vi "UHR-Fleezers Control (host) - 12.4.vi"() -> ()   [LabVIEW 2012] (continued)
                n1986 = Negate(x=w2940) -> (-x=w2941:dbl)
                n1987 = local read "Initial Y"() -> (w2947:dbl)
                n1988 = Multiply(x=w2929, y=w2938) -> (x*y=w2948:dbl)
                n1989 = Divide "X half step offset"(x=w2926, y=2.0) -> (x/y=w2934:dbl)
                n1990 = Divide "X V/pix"(x=w2926, y=w2937) -> (x/y=w2936:dbl)
                n1991 = Multiply(x=w2926, y=w2931) -> (x*y=w2943:dbl)
                n1992 = Compound Arithmetic op=ADD(w2941, w2948, w2947) -> (w2918:dbl)
                "Pointer Y (V)" <- w2918
                n1993 = Multiply(x=w2936, y=w2930) -> (x*y=w2945:dbl)
                n1994 = Negate(x=w2934) -> (-x=w2933:dbl)
                n1995 = local read "Initial X"() -> (w2946:dbl)
                n1996 = Negate(x=w2945) -> (-x=w2944:dbl)
                n1997 = Compound Arithmetic op=ADD(w2933, w2943, w2946, w2944) -> (w2919:dbl)
                "Pointer X (V)" <- w2919
                n1998 = case shown="True" "Set High F Confocal Spot (X-Y)" {
                  tunnel: w2919 -> [_ w2949]
                  tunnel: w2918 -> [_ w2950]
                  frame False {
                  }
                  frame True {
                    "Confocal Y 2 (V)" <- w2950
                    "Confocal X 2 (V)" <- w2949
                  }
                }
                n1999 = Or(x="Set X Only", y="Set Confocal Spot (X-Y)") -> (x .or. y?=w2922:bool)
                n2000 = Or(x="Set Confocal Spot (X-Y)", y="Set Y Only") -> (x .or. y?=w2921:bool)
                n2001 = case shown="True" w2922 {
                  tunnel: w2919 -> [_ w2951]
                  frame False {
                  }
                  frame True {
                    n2002 = property on="AO2" class="Slide (strict)"("Val(Sgnl)"=w2951) -> ()  [unwired: 2 in, 2 out]
                    "Confocal X 1 (V)" <- w2951
                  }
                }
                n2003 = case shown="True" w2921 {
                  tunnel: w2918 -> [_ w2952]
                  frame False {
                  }
                  frame True {
                    n2004 = property on="AO1" class="Slide (strict)"("Val(Sgnl)"=w2952) -> ()  [unwired: 2 in, 2 out]
                    "Confocal Y 1 (V)" <- w2952
                  }
                }
                n2005 = local write "Set High F Confocal Spot (X-Y)"(w2917) -> ()
                n2006 = local write "Set Confocal Spot (X-Y)"(w2917) -> ()
                n2007 = local write "Set X Only"(w2917) -> ()
                n2008 = local write "Set Y Only"(w2917) -> ()
              }
            }
          }
          frame 3 {
            n2009 = local read "BD 2 Frequency 1 (MHz)"() -> (w2953:dbl)
            n2010 = local read "BD 1 Frequency 1 (MHz)"() -> (w2954:dbl)
            n2011 = local write "Manipulating Trap"(TRUE ("Manipulating Trap")) -> ()
            n2012 = local write "Coords"(T7 {"Horizontal"=0, "Vertical"=0} ("Coords")) -> ()
            n2013 = while {
              tunnel: w2959 -> [w2964]
              tunnel: w2957 -> [w2963]
              tunnel: w2955 -> [w2962]
              tunnel: w2954 -> [w2961]
              tunnel: w2953 -> [w2960]
              stop <- w2965 stop-if-true
              n2014 = event shown="[0] \"Pane\": Mouse Move" {
                selector: _ -> [_ _]
                dyn-events: _ -> [_ _]
                timeout: _ -> [_ _]
                tunnel: ["Force Manip Abort" w3029] -> w2965
                tunnel: w2964 -> [w2972 _]
                tunnel: w2963 -> [w2970 _]
                tunnel: w2962 -> [w2969 _]
                tunnel: w2961 -> [w2968 _]
                tunnel: w2960 -> [w2967 _]
                event Mouse Move {
                  n2015 = event-data() -> ("Time"=w2973:u32, "Coords"=w2974:T7)  [unwired: 3 out]
                  n2016 = Less?(x=w2973, y=w2972) -> (x < y?=w2971:bool)
                  n2017 = case "Makes sure old motion events prior to mouse click aren't used" shown="False" w2971 {
                    tunnel: w2974 -> [w3016 _]
                    tunnel: w2970 -> [w3017 _]
                    tunnel: w2969 -> [w2994 _]
                    tunnel: w2968 -> [w2990 _]
                    tunnel: w2967 -> [w2989 _]
                    frame False {
                      n2018 = Subtract(x=w3016, y=w3017) -> (x-y=w3015:T7)
                      "Coords" <- w3015
                      n2019 = local read "Y RF Frequency Limits (MHz)"() -> (w2975:T16)
                      n2020 = To Double Precision Float(number=w3015) -> (double precision float=w3014:cluster{"Horizontal":dbl, "Vertical":dbl})
                      n2021 = Multiply(x=cluster{"Horizontal":dbl, "Vertical":dbl} {"Horizontal"=-1.0, "Vertical"=1.0}, y="Manipulation Scaling") -> (x*y=w3010:cluster{"Horizontal":dbl, "Vertical":dbl})
                      n2022 = local read "X RF Frequency Limits (MHz)"() -> (w2976:T16)
                      n2023 = Multiply(x=w3014, y=w3010) -> (x*y=w3012:cluster{"Horizontal":dbl, "Vertical":dbl})
                      n2024 = Unbundle By Name(w3012) -> ("Horizontal"=w3007:dbl, "Vertical"=w3011:dbl)
                      n2025 = Unbundle By Name(w2975) -> ("Maximum"=w2978:dbl, "Minimum"=w2977:dbl)
                      n2026 = Boolean To (0,1)(Boolean="Manip. X?") -> (0, 1=w3005:i16)
                      n2027 = Boolean To (0,1)(Boolean="Manip. Y?") -> (0, 1=w3002:i16)
                      n2028 = local read "BD 1 Frequency 2 (MHz)"() -> (w2992:dbl)
                      n2029 = Multiply(x=w3011, y=w3002) -> (x*y=w3004:dbl)
                      n2030 = Multiply(x=w3005, y=w3007) -> (x*y=w3008:dbl)
                      n2031 = local read "BD 2 Frequency 2 (MHz)"() -> (w2991:dbl)
                      n2032 = Unbundle By Name(w2976) -> ("Maximum"=w2980:dbl, "Minimum"=w2979:dbl)
                      n2033 = Add(x=w2989, y=w3004) -> (x+y=w2982:dbl)
                      n2034 = Add(x=w2990, y=w3008) -> (x+y=w2984:dbl)
                      n2035 = In Range and Coerce(upper limit=w2980, x=w2984, lower limit=w2979) -> (coerced(x)=w2983:dbl)  [unwired: 1 out]
                      n2036 = In Range and Coerce(upper limit=w2978, x=w2982, lower limit=w2977) -> (coerced(x)=w2981:dbl)  [unwired: 1 out]
                      n2037 = Subtract(x=w2983, y=w2992) -> (x-y=w3001:dbl)
                      n2038 = Subtract(x=w2981, y=w2991) -> (x-y=w3000:dbl)
                      n2039 = Square(x=w3001) -> (x^2=w2999:dbl)
                      n2040 = Square(x=w3000) -> (x^2=w2998:dbl)
                      n2041 = Add(x=w2999, y=w2998) -> (x+y=w2997:dbl)
                      n2042 = Square Root(x=w2997) -> (sqrt(x)=w2993:dbl)
                      n2043 = In Range and Coerce(upper limit="Limit Max (MHz)", x=w2993, lower limit="Limit Min (MHz)") -> (In Range?=w2986:bool)  [unwired: 1 out]
                      n2044 = Not(x="Limits Enable") -> (.not. x?=w2985:bool)
                      n2045 = Or(x=w2986, y=w2985) -> (x .or. y?=w2987:bool)
                      n2046 = case shown="True" w2987 {
                        tunnel: w2994 -> [_ w3027]
                        tunnel: w2993 -> [_ w3018]
                        tunnel: w2983 -> [_ w3025]
                        tunnel: w2992 -> [_ w3024]
                        tunnel: w2981 -> [_ w3023]
                        tunnel: w2991 -> [_ w3022]
                        tunnel: w2976 -> [_ w3020]
                        tunnel: w2975 -> [_ w3019]
                        frame False {
                        }
                        frame True {
                          n2047 = local read "BD 1 Frequency 3 (MHz)"() -> (w3026:dbl)
                          n2048 = local read "BD 2 Frequency 3 (MHz)"() -> (w3021:dbl)
                          n2049 = local write "Trap Delta (MHz)"(w3018) -> ()
                          n2050 = call "set RF board frequency - interlace.vi"("Board 2 Frequency Limits"=w3019, "Board 1 Frequency Limits"=w3020, "FPGA VI Reference In"=w3027, "Board 2 Frequency 3 (MHz)"=w3021, "Board 1 Frequency 3 (MHz)"=w3026, "Board 2 Frequency 2 (MHz)"=w3022, "Board 2 Frequency 1 (MHz)"=w3023, "Board 1 Frequency 2 (MHz)"=w3024, "Board 1 Frequency 1  (MHz)"=w3025) -> ()  [unwired: 1 in, 2 out]
                          n2051 = local write "BD 2 Frequency 1 (MHz)"(w3023) -> ()
                          n2052 = local write "BD 1 Frequency 1 (MHz)"(w3025) -> ()
                        }
                      }
                    }
                    frame True {
                    }
                  }
                }
                event Mouse Up {
                  n2053 = event-data() -> ("Button"=w3028:u16)  [unwired: 8 out]
                  n2054 = case shown="3" w3028 {
                    tunnel: [FALSE TRUE] -> w3029
                    frame 0, Default {
                    }
                    frame 3 {
                      n2055 = local read "Trap Delta (MHz)"() -> (w3031:dbl)
                      n2056 = property on="Initial delta (MHz)" class="DigNum (strict)"("Val(Sgnl)"=w3031) -> ()  [unwired: 2 in, 2 out]
                      n2057 = local write "Manipulating Trap"(FALSE ("Manipulating Trap")) -> ()
                    }
                  }
                }
              }
            }
          }
        }
      }
      event Mouse Move {
        n2058 = event-data() -> ()  [unwired: 6 out]
      }
    }
    n2059 = local read "Stop All"() -> (w2847:bool)
    n2060 = node-c288() -> ()  [unwired: 2 out]
  }
  n2061 = timed-loop "Main data acquisition loop (get data, process data for display, and save data to disk)" {
    tunnel: w12 -> [w3343]
    tunnel: w88 -> [w3342]
    tunnel: [w3372] -> w292
    tunnel: [w3367] -> w290
    timing: w200 -> [_]
    timing-out: [_] -> w199
    tunnel: w105 -> [w3196]
    stop <- "Stop All" stop-if-true
    w3113 = "Initialize"
    # "Fluorescence data into FIFO for external control vi's\n(e.g., fluorescence triggering) - Duncan Nall"
    n2062 = node-c288() -> ()  [unwired: 2 out]
    n2063 = First Call?() -> (First Call?: T/F=w3148:bool)
    n2064 = Or(x="Reset", y=w3148) -> (x .or. y?=w3149:bool)
    n2065 = local read "Flushing P1"() -> (w3068:bool)
    n2066 = case "Reset data stream (manual reset or at begining of some rastering and imaging)" shown="True" w3149 {
      tunnel: w3343 -> [w4419 w4427]
      tunnel: w3342 -> [w4418 w4426]
      tunnel: [w4419 w4421] -> w3338
      tunnel: [w4418 w4420] -> w3337
      frame False {
      }
      frame True {
        w4424 = TRUE ("AI to FIFO")
        n2067 = local write "Overflow (data lost)"(FALSE ("Overflow (data lost)")) -> ()
        n2068 = call "reset FPGA DMA.vi"("error in"=w4426, "FPGA VI Reference In"=w4427) -> ("error out"=w4422:errorcluster, "FPGA VI Reference Out"=w4423:T19)
        n2069 = xnode "Read/Write Control"("FPGA VI Reference In"=w4423, "error in"=w4422, "AI to FIFO"=w4424, "APD to FIFO"=w4424) -> ("FPGA VI Reference Out"=w4421:T19, "error out"=w4420:errorcluster)
      }
    }
    n2070 = case shown="True" w3068 {
      frame False {
      }
      frame True {
        n2071 = local read "Flush rate (uL/m) P1"() -> (w3402:dbl)
        n2072 = local read "HP1 Flush Time (s)"() -> (w3411:dbl)
        n2073 = local read "DMA Update Period (s)"() -> (w3405:dbl)
        n2074 = Divide(x=w3402, y=60.0) -> (x/y=w3403:dbl)
        n2075 = Divide(x=w3411, y=w3405) -> (x/y=w3400:dbl)
        n2076 = feedback #1(0) -> (w3409:i32)
        n2077 = Increment(x=w3409) -> (x+1=w3399:i32)
        n2078 = Greater?(x=w3399, y=w3400) -> (0:w3408:bool)
        n2079 = Compound Arithmetic op=MULTIPLY(w3405, w3399, w3403) -> (→"P1 Flush Volume (uL)":dbl)
        n2080 = Divide(x=w3399, y=w3400) -> (x/y=→"P1 Flushing Bar":dbl)
        n2081 = case shown="True" w3408 {
          tunnel: w3399 -> [w3412 _]
          tunnel: [w3412 0] -> w3407
          frame False {
          }
          frame True {
            w3413 = FALSE ("Flushing P1")
            n2082 = local write "Inject Pump 1"(w3413) -> ()
            n2083 = local write "Flushing P1"(w3413) -> ()
            n2084 = property on="Clear Volume P1" class="Bool (strict)"("Val(Sgnl)"=TRUE ("Value (Signaling)")) -> ()  [unwired: 2 in, 2 out]
          }
        }
        n2085 = feedback-in #1(w3407) -> ()
      }
    }
    n2086 = Or(x="Start AOD Scan", y="Trap Raster Scan") -> (x .or. y?=w3294:bool)
    n2087 = case "Start AOM raster scan" shown="True" w3294 {
      tunnel: w3338 -> [w4269 w4279]
      tunnel: w3337 -> [w4268 w4278]
      tunnel: [w4269 w4272] -> w3336
      tunnel: [w4268 w4271] -> w3335
      frame False {
      }
      frame True {
        n2088 = case shown="True" "Restart DMA? (AOD)" {
          tunnel: [w4317 w4319] -> w4273
          tunnel: [w4316 w4318] -> w4274
          tunnel: w4279 -> [w4317 w4321]
          tunnel: w4278 -> [w4316 w4320]
          frame False {
          }
          frame True {
            n2089 = local write "Overflow (data lost)"(FALSE ("Overflow (data lost)")) -> ()
            n2090 = call "reset FPGA DMA.vi"("error in"=w4320, "FPGA VI Reference In"=w4321) -> ("error out"=w4318:errorcluster, "FPGA VI Reference Out"=w4319:T19)
          }
        }
        n2091 = local write "Trap Raster Scan"(FALSE ("Trap Raster Scan")) -> ()
        n2092 = case shown="True" "Move MCL Also?" {
          tunnel: w4274 -> [w4282 w4311]
          tunnel: w4273 -> [w4283 w4312]
          tunnel: [w4281 w4315] -> w4272
          tunnel: [w4280 w4314] -> w4271
          frame False {
            w4284 = TRUE ("AI to FIFO")
            n2093 = xnode "Read/Write Control"("FPGA VI Reference In"=w4283, "error in"=w4282, "AI to FIFO"=w4284, "APD to FIFO"=w4284, "Start scan"=w4284) -> ("FPGA VI Reference Out"=w4281:T19, "error out"=w4280:errorcluster)
          }
          frame True {
            w4308 = FALSE ("1D or 2D Scan?")
            w4313 = TRUE ("AI to FIFO")
            # "Count for MCL loop"
            # "N total cycles"
            # "N steps"
            # "V_int"
            n2094 = local read "Scan Range (nm)"() -> (w4290:dbl)
            n2095 = local read "Number of F/B Scans (AOD)"() -> (w4307:u16)
            n2096 = Sign(1:w4290) -> (0:w4289:dbl)
            n2097 = Compound Arithmetic op=MULTIPLY(w4290, "MCL Step Position Ratio", "MCL/AOM Scale Tweak") -> (w4294:dbl)
            n2098 = Negate(x=w4289) -> (-x=w4286:dbl)
            n2099 = Multiply(x=w4286, y="MCL Step Increment (V_int)") -> (x*y=w4288:dbl)
            n2100 = Divide(x=w4294, y="MCL X Cal (nm/V)") -> (x/y=w4300:dbl)
            n2101 = Multiply(x=32767.0 ("y"), y=w4300) -> (x*y=w4306:dbl)
            n2102 = local read "Total Counts (ticks)"() -> (w4291:u16)
            n2103 = local read "Cycles/step (AOD)"() -> (w4302:u64)
            n2104 = local read "Scan steps (AOD)"() -> (w4303:u64)
            n2105 = Divide(x=w4306, y=10.0) -> (x/y=w4299:dbl)
            n2106 = Divide(x=w4299, y="MCL Step Increment (V_int)") -> (x/y=w4297:dbl)
            n2107 = Absolute Value(x=w4297) -> (abs(x)=w4285:dbl)
            n2108 = Compound Arithmetic op=MULTIPLY(w4303, w4302, w4291) -> (w4298:u64)
            n2109 = local write "wait to reset values"(w4313) -> ()
            n2110 = local write "MCL Scanning"(w4313) -> ()
            n2111 = Divide(x=w4298, y=w4285) -> (x/y=w4295:dbl)
            "MCL Count" <- w4295
            n2112 = xnode "Read/Write Control"("FPGA VI Reference In"=w4312, "error in"=w4311, "Scan steps (MCL)"=w4285, "Number of scans (MCL)"=w4307, "Cycles per step (MCL)"=u64 1, "Scan freq.  increment (MCL)"=w4288, "1D or 2D Scan?"=w4308, "MCL Scan Axis"=w4308, "Cont. Scan (MCL)"=w4308, "MCL count"=w4295) -> ("FPGA VI Reference Out"=w4310:T19, "error out"=w4309:errorcluster)
            n2113 = xnode "Read/Write Control"("FPGA VI Reference In"=w4310, "error in"=w4309, "AI to FIFO"=w4313, "APD to FIFO"=w4313, "Start scan"=w4313, "Start scan (MCL)"=w4313) -> ("FPGA VI Reference Out"=w4315:T19, "error out"=w4314:errorcluster)
          }
        }
        "Raster Scanning..." <- TRUE ("Scanning...")
      }
    }
    n2114 = local read "Flushing P3"() -> (w3069:bool)
    n2115 = case "Keep track of when Harvard Pump 3 is done flushing" shown="True" w3069 {
      frame False {
      }
      frame True {
        n2116 = local read "Flush rate (uL/m) P3"() -> (w3419:dbl)
        n2117 = local read "DMA Update Period (s)"() -> (w3421:dbl)
        n2118 = local read "HP3 Flush Time (s)"() -> (w3428:dbl)
        n2119 = Divide(x=w3419, y=60.0) -> (x/y=w3417:dbl)
        n2120 = feedback #2(0) -> (w3426:i32)
        n2121 = Increment(x=w3426) -> (x+1=w3420:i32)
        n2122 = Divide(x=w3428, y=w3421) -> (x/y=w3422:dbl)
        n2123 = Greater?(x=w3420, y=w3422) -> (0:w3425:bool)
        n2124 = Compound Arithmetic op=MULTIPLY(w3421, w3420, w3417) -> (→"P3 Flush Volume (uL)":dbl)
        n2125 = case shown="True" w3425 {
          tunnel: w3420 -> [w3429 _]
          tunnel: [w3429 0] -> w3424
          frame False {
          }
          frame True {
            w3430 = FALSE ("Flushing P3")
            n2126 = local write "Inject Pump 3"(w3430) -> ()
            n2127 = local write "Flushing P3"(w3430) -> ()
            n2128 = property on="Clear Volume P3" class="Bool (strict)"("Val(Sgnl)"=TRUE ("Value (Signaling)")) -> ()  [unwired: 2 in, 2 out]
          }
        }
        n2129 = feedback-in #2(w3424) -> ()
        n2130 = Divide(x=w3420, y=w3422) -> (x/y=→"P3 Flushing Bar":dbl)
      }
    }
    n2131 = And(x="Save scans", y=w3294) -> (x .and. y?=w3334:bool)
    n2132 = Compound Arithmetic op=OR("Start MCL Scan", "Confocal Image", "Confocal Linescan") -> (w3292:bool)
    n2133 = And(x="Save Data (MCL)", y=w3292) -> (x .and. y?=w3333:bool)
    n2134 = case "Start MCL raster scan" shown="True" w3292 {
      tunnel: w3336 -> [w3881 w3897]
      tunnel: w3335 -> [w3880 w3896]
      tunnel: [w3881 w3892] -> w3195
      tunnel: [w3880 w3891] -> w3194
      tunnel: [FALSE w3890] -> w3319
      tunnel: "Start MCL Scan" -> [_ w3885]
      tunnel: "Confocal Image" -> [_ w3884]
      tunnel: "Confocal Linescan" -> [_ _]
      frame False {
      }
      frame True {
        w3890 = TRUE
        n2135 = case shown="True" "Restart DMA? (MCL)" {
          tunnel: [w3942 w3944] -> w3895
          tunnel: [w3941 w3943] -> w3894
          tunnel: w3897 -> [w3942 w3947]
          tunnel: w3896 -> [w3941 w3946]
          frame False {
          }
          frame True {
            n2136 = call "reset FPGA DMA.vi"("error in"=w3946, "FPGA VI Reference In"=w3947) -> ("error out"=w3943:errorcluster, "FPGA VI Reference Out"=w3944:T19)
            n2137 = local write "Overflow (data lost)"(FALSE ("Overflow (data lost)")) -> ()
          }
        }
        n2138 = case shown="False" w3885 {
          selector: w3885 -> [_ w3901]
          tunnel: w3884 -> [w3900 _]
          tunnel: [w3900 w3901] -> w3883
          frame False {
            n2139 = property on="2D or 1D Scan" class="Bool (strict)"("Val(Sgnl)"=w3900) -> ()  [unwired: 2 in, 2 out]
            n2140 = property on="Confocal Image" class="Bool (strict)"("Value"=FALSE ("Start Confocal Map")) -> ()  [unwired: 2 in, 2 out]
          }
          frame True {
          }
        }
        n2141 = local write "MCL Scanning"(w3890) -> ()
        n2142 = local read "AO1"() -> (w3887:dbl)
        n2143 = local read "AO2"() -> (w3886:dbl)
        n2144 = case shown="True" "Center Scan" {
          tunnel: w3895 -> [w3908 w3940]
          tunnel: w3894 -> [w3907 w3939]
          tunnel: [w3906 w3938] -> w3892
          tunnel: [w3905 w3937] -> w3891
          tunnel: [w3903 w3924] -> w3889
          tunnel: [w3902 w3923] -> w3888
          tunnel: w3887 -> [w3903 w3929]
          tunnel: w3886 -> [w3902 w3932]
          tunnel: w3883 -> [_ _]
          frame False {
            w3904 = TRUE ("AI to FIFO")
            n2145 = xnode "Read/Write Control"("FPGA VI Reference In"=w3908, "error in"=w3907, "AI to FIFO"=w3904, "APD to FIFO"=w3904, "Start scan (MCL)"=w3904) -> ("FPGA VI Reference Out"=w3906:T19, "error out"=w3905:errorcluster)
          }
          frame True {
            w3936 = TRUE ("AI to FIFO")
            n2146 = local read "Scan steps (MCL)"() -> (w3915:u64)
            n2147 = local read "Scan lines (y)"() -> (w3911:u64)
            n2148 = local read "Fast Scan Dir"() -> (w3922:bool)
            n2149 = local read "Actual MCL Inc (V)"() -> (w3912:dbl)
            n2150 = Decrement(x=w3911) -> (x-1=w3910:u64)
            n2151 = Decrement(x=w3915) -> (x-1=w3914:u64)
            n2152 = Multiply(x=w3912, y=w3910) -> (x*y=w3909:dbl)
            n2153 = Divide(x=w3909, y=2.0) -> (x/y=w3919:dbl)
            n2154 = Multiply(x=w3912, y=w3914) -> (x*y=w3913:dbl)
            n2155 = Divide(x=w3913, y=2.0) -> (x/y=w3918:dbl)
            n2156 = Select(t=w3918, s=w3922, f=w3919) -> (s? t:f=w3917:dbl)
            n2157 = Select(t=w3919, s=w3922, f=w3918) -> (s? t:f=w3921:dbl)
            n2158 = Subtract(x=w3929, y=w3921) -> (x-y=w3920:dbl)
            n2159 = Subtract(x=w3932, y=w3917) -> (x-y=w3916:dbl)
            n2160 = local read "2D or 1D Scan"() -> (w3934:bool)
            n2161 = Not(x=w3922) -> (.not. x?=w3928:bool)
            n2162 = Not(x=w3934) -> (.not. x?=w3930:bool)
            n2163 = And(x=w3922, y=w3930) -> (x .and. y?=w3931:bool)
            n2164 = And(x=w3930, y=w3928) -> (x .and. y?=w3933:bool)
            n2165 = Select(t=w3932, s=w3933, f=w3916) -> (s? t:f=w3923:dbl)
            n2166 = Select(t=w3929, s=w3931, f=w3920) -> (s? t:f=w3924:dbl)
            n2167 = call "Volt to I16.vi"("Voltage In"=w3924) -> ("I16 Voltage Out"=w3927:i16)
            n2168 = call "Volt to I16.vi"("Voltage In"=w3923) -> ("I16 Voltage Out"=w3926:i16)
            n2169 = xnode "Read/Write Control"("FPGA VI Reference In"=w3940, "error in"=w3939, "AI to FIFO"=w3936, "APD to FIFO"=w3936, "Start scan (MCL)"=w3936, "AO1"=w3927, "AO2"=w3926) -> ("FPGA VI Reference Out"=w3938:T19, "error out"=w3937:errorcluster)
          }
        }
        "Initial Y" <- w3889
        "Initial X" <- w3888
        n2170 = local write "Tab Control 6"(T3."Imaging" ("Tab Control 6")) -> ()
        "wait to reset values" <- w3890
      }
    }
    n2171 = local read "APD Elements/DMA read"() -> (w3036:u32)
    n2172 = local read "Trap AI Elements/DMA read"() -> (w3257:u32)
    n2173 = xnode "Get APD Data"("FPGA VI Reference In"=w3195, "error in"=w3194, "Number of Elements"=w3036, "Timeout (ms)"=-1) -> ("Data"=w3226:u32[], "Elements Remaining"=→"APD FIFO Elements Remaining":u32)  [unwired: 2 out]
    n2174 = local read "Trap Pos Elements/DMA read"() -> (w3191:u32)
    n2175 = xnode "Invoke Method"("FPGA VI Reference In"=w3195, "error in"=w3194, "Number of Elements"=w3191, "Timeout (ms)"=-1) -> ("Data"=w3155:u16[], "Elements Remaining"=→"Trap Pos FIFO El Remaining":u32)  [unwired: 2 out]
    n2176 = xnode "Get Trap Data"("FPGA VI Reference In"=w3195, "error in"=w3194, "Number of Elements"=w3257, "Timeout (ms)"=-1 ("Timeout")) -> ("FPGA VI Reference Out"=w3090:T19, "error out"=w3089:errorcluster, "Data"=w3156:i16[], "Elements Remaining"=w3380:u32)
    "FIFO El. Rem." <- w3380
    n2177 = local read "DMA Update Period (s)"() -> (w3258:dbl)
    n2178 = local read "Trap AI FIFO Depth"() -> (w3382:u32)
    n2179 = local read "Number of APDs"() -> (w3058:u8)
    n2180 = Decimate 1D Array(w3155) -> (w3152:u16[], w3154:u16[], w3153:u16[])
    n2181 = feedback #3(0.0) -> (w3184:dbl)
    n2182 = Add(x=w3258, y=w3184) -> (x+y=w3356:dbl)
    n2183 = feedback-in #3(w3356) -> ()
    n2184 = To Time Stamp(1:w3184) -> (0:w3183:timestamp)
    n2185 = Subtract(x=w3382, y=w3257) -> (x-y=w3381:u32)
    n2186 = To Unsigned Long Integer(number=w3152) -> (unsigned 32bit integer=w3151:u32[])
    n2187 = Join Numbers(hi=w3154, lo=w3153) -> ((hi.lo)=w3150:u32[])
    n2188 = Divide(x=w3380, y=w3381) -> (x/y=w3379:dbl)
    "Buffer Status" <- w3379
    n2189 = case "Deinterlace APD signals" shown="3, Default" w3058 {
      tunnel: [w3392 w3398] -> w3035
      tunnel: w3226 -> [w3393 w3397]
      tunnel: [w3391 w3396] -> w3034
      tunnel: [w3390 w3394] -> w3041
      frame 3, Default {
        n2190 = Decimate 1D Array "APD signals"(w3393) -> (w3392:u32[], w3391:u32[], w3390:u32[])
      }
      frame 2 {
        n2191 = Decimate 1D Array "APD signals"(w3397) -> (w3398:u32[], w3396:u32[])
        n2192 = Multiply(x=w3396, y=u32 0) -> (x*y=w3394:u32[])
      }
    }
    n2193 = Join Numbers(hi=w3151, lo=w3150) -> ((hi.lo)=w3144:u64[])
    n2194 = call "IR AOM word to freq - vec.vi"("Frequency Word In (double vec)"=w3144) -> ("Frequency Out"=w3190:dbl[])
    n2195 = Equal?(x=w3379, y=1.0) -> (x = y?=w3377:bool)
    n2196 = case "Alert buffer overflow" shown="True" w3377 {
      frame False {
      }
      frame True {
        n2197 = call <vilib>:"Beep.vi"() -> ()  [unwired: 3 in, 9 out]
        "Overflow (data lost)" <- TRUE ("Overflow (data lost)")
      }
    }
    n2198 = Decimate 1D Array(w3190) -> (w3189:dbl[], w3188:dbl[])
    n2199 = Build Array(w3189, w3188) -> (w3187:dbl[][])
    n2200 = Bundle(w3035, w3034, w3041) -> (w3039:cluster{u32[], u32[], u32[]})  [unwired: 1 in]
    n2201 = Build Array(w3035, w3034, w3041) -> (w3316:u32[][])
    n2202 = for {
      tunnel: w3035 -> [w3388] mode=indexing
      n2203 = call "Smart Buffer (DBL) 1.vi"("new element [write]"=w3388, "mode"=T20."write") -> ()  [unwired: 4 in, 6 out]
    }
    n2204 = local read "APD Integration Time (s)"() -> (w3051:dbl)
    n2205 = To Double Precision Float(number=w3316) -> (double precision float=w3317:dbl[][])
    n2206 = feedback #4 "APD3"(w3041) -> (w3057:u32[])
    n2207 = feedback #5 "APD2"(w3034) -> (w3213:u32[])
    n2208 = feedback #6 "APD1"(w3035) -> (w3315:u32[])
    n2209 = Build Array (concatenate)(w3213, w3034) -> (w3212:u32[])
    n2210 = Build Array (concatenate)(w3057, w3041) -> (w3056:u32[])
    n2211 = Build Array (concatenate)(w3315, w3035) -> (w3312:u32[])
    n2212 = for {
      tunnel: w3034 -> [w3387] mode=indexing
      n2213 = call "Smart Buffer (DBL) 2.vi"("new element [write]"=w3387, "mode"=T20."write") -> ()  [unwired: 4 in, 6 out]
    }
    n2214 = Array Size(array=w3312) -> (size(s)=w3309:i32)
    n2215 = Array Size(array=w3035) -> (size(s)=w3311:i32)
    n2216 = Multiply(x=w3311, y="APD Ave N") -> (x*y=w3310:dbl)
    n2217 = Greater?(x=w3309, y=w3310) -> (0:w3313:bool)
    n2218 = Bundle("APD 1", "APD 2", "APD 3") -> (w3349:cluster{string, string, string})  [unwired: 1 out]
    n2219 = local read "Trap Sets"() -> (w3256:u32)
    n2220 = case shown="True" w3313 {
      tunnel: w3312 -> [w3696 w3705]
      tunnel: [w3696 w3703] -> w3263
      tunnel: w3310 -> [_ w3698]
      tunnel: w3309 -> [_ w3704]
      tunnel: w3212 -> [w3695 w3702]
      tunnel: [w3695 w3701] -> w3210
      tunnel: w3056 -> [w3694 w3700]
      tunnel: [w3694 w3697] -> w3052
      frame False {
      }
      frame True {
        n2221 = Subtract(x=w3704, y=w3698) -> (x-y=w3699:dbl)
        n2222 = Array Subset "APD3"(array=w3700, index=w3699, length=w3698) -> (w3697:u32[])
        n2223 = Array Subset "APD2"(array=w3702, index=w3699, length=w3698) -> (w3701:u32[])
        n2224 = Array Subset "APD1"(array=w3705, index=w3699, length=w3698) -> (w3703:u32[])
      }
    }
    n2225 = feedback-in #4(w3052) -> ()
    n2226 = feedback-in #5(w3210) -> ()
    n2227 = feedback-in #6(w3263) -> ()
    n2228 = Cluster To Array(cluster=w3349) -> (array=w3346:string[])
    n2229 = for "APD" {
      tunnel: w3317 -> [w3952] mode=indexing
      tunnel: w3051 -> [w3959]
      tunnel: [w3955] -> w3214 mode=indexing
      tunnel: "APD Disp. Scale" -> [w3956]
      tunnel: w3346 -> [w3954] mode=indexing
      tunnel: "APD Disp. Downsample" -> [w3950]
      tunnel: [w3953] -> w3345
      workers-P: _ -> [_]
      tunnel: w3183 -> [w3949]
      n2230 = call "integrate 1D array interval - double.vi"("Ave N"=w3950, "Array In"=w3952) -> ("Array Out"=w3951:dbl[])  [unwired: 1 out]
      n2231 = Multiply(x=w3959, y=w3950) -> (x*y=w3953:dbl)
      n2232 = Divide(x=w3951, y=w3956) -> (x/y=w3957:dbl[])
      n2233 = Bundle By Name("t0"=w3949, "Y"=w3957, "dt"=w3953) -> (w3958:waveform(dbl))  [unwired: 1 out]
      n2234 = Set Waveform Attribute(5:w3954, 6:"NI_ChannelName" ("name"), 7:w3958) -> (3:w3955:waveform(dbl))  [unwired: 1 in, 2 out]
    }
    "APD Display Period (s)" <- w3345
    n2235 = Reciprocal(x=w3345) -> (1/x=→"APD Display Freq. (Hz)":dbl)
    n2236 = case "Deinterlace trap data, average down PSD" shown="2" w3256 {
      tunnel: w3156 -> [w3977 w4042]
      tunnel: [w3974 w4039] -> w3249
      tunnel: [w3977 w4041] -> w3147
      tunnel: "Detector Type" -> [w3976 w4037]
      tunnel: [w3975 w4040] -> w3248
      tunnel: [w3973 w4038] -> w3354
      frame 1, Default {
        n2237 = Divide(x=w3977, y=3276.7) -> (x/y=w3978:dbl[])
        n2238 = Decimate 1D Array(w3978) -> (w3987:dbl[], w3986:dbl[], w3985:dbl[], w3984:dbl[], w3983:dbl[], w3982:dbl[], w3981:dbl[], w3980:dbl[])
        n2239 = case shown="\"IR-QPD + PSD + FB-QPD position\"" w3976 {
          tunnel: w3987 -> [w4011 w4036]
          tunnel: w3986 -> [w4010 w4035]
          tunnel: w3985 -> [w3995 w4013]
          tunnel: w3984 -> [w3996 w4023]
          tunnel: w3983 -> [w4009 w4034]
          tunnel: w3982 -> [w4008 w4033]
          tunnel: w3981 -> [w3992 w4014]
          tunnel: w3980 -> [w3991 w4012]
          tunnel: [w3990 w4020] -> w3975
          tunnel: [w3989 w4019] -> w3974
          tunnel: [w3988 w4018] -> w3973
          frame "IR-QPD + PSD + FB-QPD", Default {
            w3988 = 0  # Channel pattern
            n2240 = Divide(x=w4011, y=w3996) -> (x/y=w3998:dbl[])
            n2241 = Divide(x=w4010, y=w3996) -> (x/y=w3997:dbl[])
            n2242 = Divide(x=w4009, y=w3992) -> (x/y=w3994:dbl[])
            n2243 = Divide(x=w4008, y=w3991) -> (x/y=w3993:dbl[])
            n2244 = Build Array(w3998, w3997, w3996, w3995, w3994, w3993, w3992, w3991) -> (w3989:dbl[][])
            n2245 = Bundle("T1 Y", "T1 X", "T1 Sum", "FB Sum", "PSD Y", "PSD X", "PSD Y Sum", "PSD X Sum") -> (w4007:T39)  [unwired: 1 out]
            n2246 = Cluster To Array(cluster=w4007) -> (array=w3990:string[])
          }
          frame "IR-QPD + PSD + FB-QPD position" {
            w4018 = 3  # Channel pattern
            n2247 = Negate(x=w4014) -> (-x=w4015:dbl[])
            n2248 = Divide(x=w4036, y=w4023) -> (x/y=w4025:dbl[])
            n2249 = Divide(x=w4035, y=w4023) -> (x/y=w4024:dbl[])
            n2250 = Divide(x=w4034, y=w4014) -> (x/y=w4022:dbl[])
            n2251 = Divide(x=w4033, y=w4015) -> (x/y=w4021:dbl[])
            n2252 = Build Array(w4025, w4024, w4023, w4012, w4013, w4022, w4021, w4014) -> (w4019:dbl[][])
            n2253 = Bundle("T1 Y", "T1 X", "T1 Sum", "FB X", "FB Sum", "PSD Y", "PSD X", "PSD Y Sum") -> (w4032:T39)  [unwired: 1 out]
            n2254 = Cluster To Array(cluster=w4032) -> (array=w4020:string[])
          }
        }
      }
      frame 2 {
        n2255 = case shown="\"IR-QPD + PSD + FB-QPD X position\"" w4037 {
          tunnel: w4042 -> [w4104 w4176 w4247]
          tunnel: [w4043 w4167 w4178] -> w4041
          tunnel: [w4070 w4158 w4225] -> w4040
          tunnel: [w4069 w4121 w4192] -> w4039
          tunnel: [w4063 w4156 w4223] -> w4038
          frame "IR-QPD + PSD + FB-QPD", Default {
            w4063 = 1  # Channel pattern
            # "time average x2 the 4th signal and the 4 psd signals (detection laser)"
            # "deinterlace 3 signals from qpd"
            n2256 = Decimate 1D Array(w4104) -> (w4103:i16[], w4102:i16[], w4068:i16[], w4101:i16[], w4091:i16[], w4089:i16[], w4088:i16[], w4086:i16[])
            n2257 = Decimate 1D Array(w4068) -> (w4067:i16[], w4066:i16[])
            n2258 = Decimate 1D Array(w4103) -> (w4100:i16[], w4072:i16[])
            n2259 = Decimate 1D Array(w4102) -> (w4099:i16[], w4097:i16[])
            n2260 = Decimate 1D Array(w4101) -> (w4098:i16[], w4096:i16[])
            n2261 = call "downsample 1D array - double.vi"("Ave N"=2.0, "Array In"=w4091) -> ("Array Out"=w4090:dbl[])  [unwired: 1 out]
            n2262 = call "downsample 1D array - double.vi"("Ave N"=2.0, "Array In"=w4089) -> ("Array Out"=w4071:dbl[])  [unwired: 1 out]
            n2263 = call "downsample 1D array - double.vi"("Ave N"=2.0, "Array In"=w4088) -> ("Array Out"=w4087:dbl[])  [unwired: 1 out]
            n2264 = call "downsample 1D array - double.vi"("Ave N"=2.0, "Array In"=w4086) -> ("Array Out"=w4085:dbl[])  [unwired: 1 out]
            n2265 = Interleave 1D Arrays(w4100, w4099, w4098, w4072, w4097, w4096, w4067, w4066, w4090, w4071, w4087, w4085) -> (w4084:dbl[])
            n2266 = Divide(x=w4084, y=3276.7) -> (x/y=w4083:dbl[])
            n2267 = Decimate 1D Array(w4083) -> (w4082:dbl[], w4081:dbl[], w4080:dbl[], w4079:dbl[], w4078:dbl[], w4077:dbl[], w4065:dbl[], w4064:dbl[], w4076:dbl[], w4075:dbl[], w4074:dbl[], w4073:dbl[])
            n2268 = Divide(x=w4082, y=w4080) -> (x/y=w4050:dbl[])
            n2269 = Divide(x=w4081, y=w4080) -> (x/y=w4049:dbl[])
            n2270 = Divide(x=w4079, y=w4077) -> (x/y=w4048:dbl[])
            n2271 = Divide(x=w4078, y=w4077) -> (x/y=w4047:dbl[])
            n2272 = Divide(x=w4076, y=w4074) -> (x/y=w4046:dbl[])
            n2273 = Divide(x=w4075, y=w4073) -> (x/y=w4045:dbl[])
            n2274 = Build Array(w4050, w4049, w4080, w4048, w4047, w4077, w4065, w4064, w4046, w4045, w4074, w4073) -> (w4069:dbl[][])
            n2275 = Bundle("T1 Y", "T1 X", "T1 Sum", "T2 Y", "T2 X", "T2 Sum", "T1 FB Sum", "T2 FB Sum", "PSD Y", "PSD X", "PSD Y Sum", "PSD X Sum") -> (w4051:T40)  [unwired: 1 out]
            n2276 = To Word Integer(number=w4084) -> (16bit integer=w4043:i16[])
            n2277 = Cluster To Array(cluster=w4051) -> (array=w4070:string[])
          }
          frame "IR-QPD + PSD + FB-QPD X position" {
            w4156 = 2  # Channel pattern
            # "time average x2 the 3 psd signals (detection laser)"
            # "deinterlace 3 signals from qpds"
            n2278 = Decimate 1D Array(w4176) -> (w4175:i16[], w4174:i16[], w4157:i16[], w4173:i16[], w4119:i16[], w4116:i16[], w4113:i16[], w4144:i16[])
            n2279 = Select(t=i16 -1, s="Flip X Sign", f=i16 1) -> (s? t:f=w4109:i16)
            n2280 = Multiply(x=w4174, y=w4109) -> (x*y=w4110:i16[])
            n2281 = Decimate 1D Array(w4157) -> (w4142:i16[], w4140:i16[])
            n2282 = Decimate 1D Array(w4175) -> (w4172:i16[], w4159:i16[])
            n2283 = Decimate 1D Array(w4110) -> (w4171:i16[], w4169:i16[])
            n2284 = Decimate 1D Array(w4173) -> (w4170:i16[], w4168:i16[])
            n2285 = Decimate 1D Array(w4144) -> (w4143:i16[], w4141:i16[])
            n2286 = call "downsample 1D array - I16.vi"("Ave N"=2.0, "Array In"=w4119) -> ("Array Out"=w4117:i16[])  [unwired: 1 in]
            n2287 = call "downsample 1D array - I16.vi"("Ave N"=2.0, "Array In"=w4113) -> ("Array Out"=w4111:i16[])  [unwired: 1 in]
            n2288 = call "downsample 1D array - I16.vi"("Ave N"=2.0, "Array In"=w4116) -> ("Array Out"=w4114:i16[])  [unwired: 1 in]
            n2289 = Interleave 1D Arrays(w4172, w4171, w4170, w4159, w4169, w4168, w4143, w4142, w4141, w4140, w4117, w4114, w4111) -> (w4167:i16[])
            n2290 = Divide(x=w4167, y=3276.7) -> (x/y=w4166:dbl[])
            n2291 = Decimate 1D Array(w4166) -> (w4165:dbl[], w4164:dbl[], w4163:dbl[], w4162:dbl[], w4161:dbl[], w4160:dbl[], w4132:dbl[], w4130:dbl[], w4129:dbl[], w4127:dbl[], w4126:dbl[], w4125:dbl[], w4122:dbl[])
            n2292 = Negate(x=w4122) -> (-x=w4120:dbl[])
            n2293 = Divide(x=w4126, y=w4122) -> (x/y=w4124:dbl[])
            n2294 = Divide(x=w4125, y=w4120) -> (x/y=w4123:dbl[])
            n2295 = Divide(x=w4165, y=w4163) -> (x/y=w4148:dbl[])
            n2296 = Divide(x=w4164, y=w4163) -> (x/y=w4147:dbl[])
            n2297 = Divide(x=w4162, y=w4160) -> (x/y=w4146:dbl[])
            n2298 = Divide(x=w4161, y=w4160) -> (x/y=w4145:dbl[])
            n2299 = Divide(x=w4132, y=w4130) -> (x/y=w4131:dbl[])
            n2300 = Divide(x=w4129, y=w4127) -> (x/y=w4128:dbl[])
            n2301 = Build Array(w4148, w4147, w4163, w4146, w4145, w4160, w4131, w4130, w4128, w4127, w4124, w4123, w4122) -> (w4121:dbl[][])
            n2302 = Bundle("T1 Y", "T1 X", "T1 Sum", "T2 Y", "T2 X", "T2 Sum", "T1 FB X", "T1 FB Sum", "T2 FB X", "T2 FB Sum", "PSD Y", "PSD X", "PSD Y Sum") -> (w4149:T41)  [unwired: 1 out]
            n2303 = Cluster To Array(cluster=w4149) -> (array=w4158:string[])
          }
          frame "IR-QPD + PSD + FB-QPD XY positions" {
            w4223 = 4  # Channel pattern
            # "time average x2 the 3 psd signals (detection laser)"
            # "deinterlace 3 signals from qpds"
            n2304 = Decimate 1D Array(w4247) -> (w4246:i16[], w4245:i16[], w4224:i16[], w4244:i16[], w4190:i16[], w4236:i16[], w4235:i16[], w4212:i16[])
            n2305 = Decimate 1D Array "Feedback Sum"(w4224) -> (w4208:i16[], w4206:i16[])
            n2306 = Decimate 1D Array "QPD Y"(w4246) -> (w4243:i16[], w4226:i16[])
            n2307 = Decimate 1D Array "QPD X"(w4245) -> (w4242:i16[], w4240:i16[])
            n2308 = Decimate 1D Array "Feedback Y"(w4190) -> (w4189:i16[], w4188:i16[])
            n2309 = Decimate 1D Array "QPD Sum"(w4244) -> (w4241:i16[], w4239:i16[])
            n2310 = Decimate 1D Array "Feedback X"(w4212) -> (w4209:i16[], w4207:i16[])
            n2311 = call "downsample 1D array - double.vi"("Ave N"=2.0, "Array In"=w4236) -> ("Array Out"=w4211:dbl[])  [unwired: 1 out]
            n2312 = call "downsample 1D array - double.vi"("Ave N"=2.0, "Array In"=w4235) -> ("Array Out"=w4210:dbl[])  [unwired: 1 out]
            n2313 = Interleave 1D Arrays(w4243, w4242, w4241, w4226, w4240, w4239, w4189, w4209, w4208, w4188, w4207, w4206, w4211, w4210) -> (w4234:dbl[])
            n2314 = Divide(x=w4234, y=3276.7) -> (x/y=w4233:dbl[])
            n2315 = Decimate 1D Array(w4233) -> (w4232:dbl[], w4231:dbl[], w4230:dbl[], w4229:dbl[], w4228:dbl[], w4227:dbl[], w4185:dbl[], w4199:dbl[], w4183:dbl[], w4184:dbl[], w4197:dbl[], w4181:dbl[], w4195:dbl[], w4193:dbl[])
            n2316 = Negate(x=w4193) -> (-x=w4191:dbl[])
            n2317 = Divide(x=w4195, y=w4191) -> (x/y=w4194:dbl[])
            n2318 = Divide(x=w4184, y=w4181) -> (x/y=w4180:dbl[])
            n2319 = Divide(x=w4185, y=w4183) -> (x/y=w4182:dbl[])
            n2320 = Divide(x=w4232, y=w4230) -> (x/y=w4216:dbl[])
            n2321 = Divide(x=w4231, y=w4230) -> (x/y=w4215:dbl[])
            n2322 = Divide(x=w4229, y=w4227) -> (x/y=w4214:dbl[])
            n2323 = Divide(x=w4228, y=w4227) -> (x/y=w4213:dbl[])
            n2324 = Divide(x=w4199, y=w4183) -> (x/y=w4198:dbl[])
            n2325 = Divide(x=w4197, y=w4181) -> (x/y=w4196:dbl[])
            n2326 = Build Array(w4216, w4215, w4230, w4214, w4213, w4227, w4182, w4198, w4183, w4180, w4196, w4181, w4194, w4193) -> (w4192:dbl[][])
            n2327 = Bundle("T1 Y", "T1 X", "T1 Sum", "T2 Y", "T2 X", "T2 Sum", "T1 FB Y", "T1 FB X", "T1 FB Sum", "T2 FB Y", "T2 FB X", "T2 FB Sum", "PSD X", "PSD Y Sum") -> (w4179:T42)  [unwired: 1 out]
            n2328 = To Word Integer(number=w4234) -> (16bit integer=w4178:i16[])
            n2329 = Cluster To Array(cluster=w4179) -> (array=w4225:string[])
          }
        }
      }
    }
    "AI labels" <- w3248
    n2330 = local read "APD Integration Time (s)"() -> (w3221:dbl)
    n2331 = Array Size(array=w3263) -> (size(s)=w3308:i32)
    n2332 = call <vilib>:"Std Deviation and Variance.vi"("X"=w3210) -> ("standard deviation"=w3209:dbl)  [unwired: 1 in, 2 out]
    n2333 = Add Array Elements(numeric array=w3210) -> (sum=w3211:u32)
    n2334 = Add Array Elements(numeric array=w3263) -> (sum=w3318:u32)
    n2335 = call <vilib>:"Std Deviation and Variance.vi"("X"=w3263) -> ("standard deviation"=w3262:dbl)  [unwired: 1 in, 2 out]
    n2336 = Divide(x=w3209, y=w3051) -> (x/y=w3206:dbl)
    "Rate sigma (Hz) 2" <- w3206
    n2337 = Multiply(x=w3051, y=w3308) -> (x*y=w3053:dbl)
    "Int. Time (s)" <- w3053
    n2338 = Divide(x=w3211, y=w3053) -> (x/y=w3207:dbl)
    "APD 2 Rate (Hz)" <- w3207
    n2339 = Multiply(x="APD Disp. Scale", y=w3214) -> (x*y=w3223:waveform(dbl)[])
    n2340 = Divide(x=w3318, y=w3053) -> (x/y=w3260:dbl)
    "APD 1 Rate (Hz)" <- w3260
    n2341 = Divide(x=w3262, y=w3051) -> (x/y=w3261:dbl)
    "Rate sigma (Hz)" <- w3261
    n2342 = Divide(x=w3206, y=w3207) -> (x/y=→"Sigma/Mean 2":dbl)
    n2343 = Multiply(x="APD Disp. Downsample", y=w3221) -> (x*y=w3219:dbl)
    n2344 = Divide(x=w3261, y=w3260) -> (x/y=→"Sigma/Mean":dbl)
    n2345 = Divide(x=w3223, y=w3219) -> (x/y=w3043:waveform(dbl)[])
    n2346 = Index Array(array=w3043, index=0) -> (element=w3203:waveform(dbl))
    n2347 = Index Array(array=w3043, index=1) -> (element=w3201:waveform(dbl))
    n2348 = Index Array(array=w3043, index=2) -> (element=w3045:waveform(dbl))
    n2349 = Subtract(x=w3203, y="APD 1 Offset") -> (x-y=w3199:waveform(dbl))
    n2350 = Subtract(x=w3201, y="APD 2 Offset") -> (x-y=w3198:waveform(dbl))
    n2351 = Subtract(x=w3045, y="APD 3 Offset") -> (x-y=w3042:waveform(dbl))
    n2352 = Add Array Elements(numeric array=w3052) -> (sum=w3055:u32)
    n2353 = call <vilib>:"Std Deviation and Variance.vi"("X"=w3052) -> ("standard deviation"=w3054:dbl)  [unwired: 1 in, 2 out]
    n2354 = Build Array(w3199, w3198, w3042) -> (→"APD Chart":waveform(dbl)[])
    n2355 = Divide(x=w3055, y=w3053) -> (x/y=w3049:dbl)
    "APD 3 Rate (Hz)" <- w3049
    n2356 = Divide(x=w3054, y=w3051) -> (x/y=w3050:dbl)
    "Rate sigma (Hz) 3" <- w3050
    n2357 = Divide(x=w3050, y=w3049) -> (x/y=→"Sigma/Mean 3":dbl)
    n2358 = local read "Data Period (s)"() -> (w3106:dbl)
    n2359 = local read "BD 1 Frequency 2 (MHz)"() -> (w3139:dbl)
    n2360 = local read "BD 1 Frequency 1 (MHz)"() -> (w3140:dbl)
    n2361 = Decimate 1D Array(w3147) -> (w3171:i16[], w3170:i16[], w3168:i16[], w3167:i16[])  [unwired: 9 out]
    n2362 = Multiply(x=w3106, y="Trap Pos. Disp. Downsample") -> (x*y=w3104:dbl)
    n2363 = Divide(x=w3171, y=w3170) -> (x/y=w3172:dbl[])
    n2364 = Divide(x=w3168, y=w3167) -> (x/y=w3169:dbl[])
    n2365 = local read "AOM X Cal (nm/MHz)"() -> (w3137:dbl)
    n2366 = Split 1D Array(array=w3172, index="N El. to Ave.") -> (second subarray=w3175:dbl[])  [unwired: 1 out]
    n2367 = Split 1D Array(array=w3169, index="N El. to Ave.") -> (second subarray=w3174:dbl[])  [unwired: 1 out]
    n2368 = Multiply(x=w3106, y="Trap Disp. Downsample") -> (x*y=w3185:dbl)
    "Display Period (s)" <- w3185
    n2369 = for "Trap AI" {
      tunnel: [w3972] -> w3350 mode=indexing
      tunnel: w3183 -> [w3963]
      tunnel: "Trap Disp. Downsample" -> [w3970]
      tunnel: w3249 -> [w3968] mode=indexing
      tunnel: w3106 -> [w3967]
      tunnel: w3248 -> [w3966] mode=indexing
      tunnel: [w3965] -> w3218 mode=indexing
      tunnel: w3185 -> [w3964]
      workers-P: _ -> [_]
      n2370 = Bundle By Name("Y"=w3968, "dt"=w3967) -> (w3969:waveform(dbl))  [unwired: 1 out]
      n2371 = Set Waveform Attribute(5:w3966, 6:"NI_ChannelName" ("name"), 7:w3969) -> (3:w3965:waveform(dbl))  [unwired: 1 in, 2 out]
      n2372 = call "downsample 1D array - double.vi"("Ave N"=w3970, "Array In"=w3968) -> ("Array Out"=w3971:dbl[])  [unwired: 1 out]
      n2373 = Bundle By Name(cluster=w3965, "t0"=w3963, "Y"=w3971, "dt"=w3964) -> (w3972:waveform(dbl))
    }
    n2374 = Bundle("BD 1 Frequency 1 (MHz)"=w3140, "BD 1 Frequency 2 (MHz)"=w3139) -> (w3141:T43)  [unwired: 1 out]
    n2375 = call-poly <vilib>:"Mean.vi"("X"=w3174) -> ("mean"=w3162:dbl)  [unwired: 1 out]
    n2376 = call-poly <vilib>:"Mean.vi"("X"=w3175) -> ("mean"=w3163:dbl)  [unwired: 1 out]
    n2377 = Reciprocal(x=w3185) -> (1/x=→"Trap Disp. Freq. (Hz)":dbl)
    n2378 = Cluster To Array(cluster=w3141) -> (array=w3138:dbl[])
    n2379 = local read "Trap X AI1 (DMA)"() -> (w3173:T13)
    n2380 = local read "Data points/scans (MCL)"() -> (w3328:dbl)
    n2381 = To Fixed-Point(number=w3162) -> (fixed-point=w3160:fxp<+/-,16,1>)  [unwired: 1 in]
    n2382 = To Fixed-Point(number=w3163) -> (fixed-point=w3161:fxp<+/-,16,1>)  [unwired: 1 in]
    n2383 = Bundle("Trap 1 Pos.", "Trap 2 Pos.") -> (w3182:cluster{string, string})  [unwired: 1 out]
    n2384 = Bundle By Name(cluster=w3173, "Set 1"=w3161, "Set 2"=w3160) -> (→"Trap X AI1 (DMA)":T13)
    n2385 = Cluster To Array(cluster=w3182) -> (array=w3179:string[])
    n2386 = Unbundle(w3039) -> (w3040:u32[])  [unwired: 2 out]
    n2387 = Select(t=-1.0, s="Negate Y Axis", f=1.0) -> (s? t:f=w3123:dbl)
    n2388 = for "Trap Position" {
      tunnel: w3187 -> [w3558] mode=indexing
      tunnel: "Trap Pos. Disp. Downsample" -> [w3557]
      tunnel: w3104 -> [w3555]
      tunnel: w3183 -> [w3554]
      tunnel: w3179 -> [w3552] mode=indexing
      tunnel: [w3551] -> w3093 mode=indexing
      tunnel: w3138 -> [w3549] mode=indexing
      tunnel: w3137 -> [w3547]
      tunnel: w3123 -> [w3546]
      n2389 = call "downsample 1D array - double.vi"("Ave N"=w3557, "Array In"=w3558) -> ("Array Out"=w3556:dbl[])  [unwired: 1 out]
      n2390 = Subtract(x=w3556, y=w3549) -> (x-y=w3550:dbl[])
      n2391 = Multiply(x=w3547, y=w3550) -> (x*y=w3548:dbl[])
      n2392 = Multiply(x=w3546, y=w3548) -> (x*y=w3545:dbl[])
      n2393 = Bundle By Name("Y"=w3545, "dt"=w3555, "t0"=w3554) -> (w3553:waveform(dbl))  [unwired: 1 out]
      n2394 = Set Waveform Attribute(5:w3552, 6:"NI_ChannelName" ("name"), 7:w3553) -> (3:w3551:waveform(dbl))  [unwired: 1 in, 2 out]
    }
    n2395 = To Double Precision Float(number=w3040) -> (double precision float=w3246:dbl[])
    n2396 = local read "Display Period (s)"() -> (w3235:dbl)
    n2397 = Increment(x=w3328) -> (x+1=w3329:dbl)
    n2398 = Index Array(array=w3093, index=0) -> (element=w3097:waveform(dbl))
    n2399 = Index Array(array=w3093, index=1) -> (element=w3092:waveform(dbl))
    n2400 = feedback #7(w3329) -> (w3332:dbl)
    n2401 = Select(t=0, s=w3319, f=w3332) -> (s? t:f=w3325:dbl)
    n2402 = Array Size(array=w3246) -> (size(s)=w3331:i32)
    n2403 = Build Array (concatenate)(w3214, w3350) -> (w3216:waveform(dbl)[])
    "All Signals" <- w3216
    n2404 = Add(x=w3331, y=w3325) -> (x+y=w3326:dbl)
    n2405 = Unbundle By Name(w3097) -> ("Y"=w3098:dbl[])
    n2406 = Divide(x="Bead Sep. Int. Time (s)", y=w3235) -> (x/y=w3133:dbl)
    n2407 = Add(x=w3098, y="FB Trap Pos Offset") -> (x+y=w3096:dbl[])
    "T1 x pos data" <- w3096
    n2408 = Greater?(x=w3326, y=w3328) -> (0:w3327:bool)
    n2409 = feedback #8(w3096) -> (w3135:dbl[])
    n2410 = Build Array (concatenate)(w3096, w3135) -> (w3134:dbl[])
    n2411 = Bundle By Name(cluster=w3097, "Y"=w3096) -> (w3095:waveform(dbl))
    n2412 = Select(t=w3325, s=w3327, f=w3326) -> (s? t:f=w3324:dbl)
    n2413 = feedback-in #7(w3324) -> ()
    n2414 = local read "MCL Scanning"() -> (w3322:bool)
    n2415 = Bundle(w3095, w3092) -> (w3091:cluster{waveform(dbl), waveform(dbl)})  [unwired: 1 out]
    n2416 = Split 1D Array(array=w3134, index=w3133) -> (first subarray=w3127:dbl[])  [unwired: 1 out]
    n2417 = feedback-in #8(w3127) -> ()
    n2418 = Not(x=w3327) -> (.not. x?=w3321:bool)
    n2419 = Cluster To Array(cluster=w3091) -> (array=w3067:waveform(dbl)[])
    "Trap Positions" <- w3067
    n2420 = call-poly <vilib>:"Mean.vi"("X"=w3127) -> ("mean"=w3126:dbl)  [unwired: 1 out]
    "Mean T1 Position (nm)" <- w3126
    n2421 = Subtract(x=w3127, y=w3126) -> (x-y=w3132:dbl[])
    n2422 = Square(x=w3132) -> (x^2=w3131:dbl[])
    n2423 = And(x=w3321, y=w3322) -> (x .and. y?=w3323:bool)
    n2424 = call-poly <vilib>:"Mean.vi"("X"=w3131) -> ("mean"=w3130:dbl)  [unwired: 1 out]
    n2425 = Square Root(x=w3130) -> (sqrt(x)=w3129:dbl)
    n2426 = Or(x=w3323, y=w3319) -> (x .or. y?=w3320:bool)
    n2427 = Equal?(x="Tab Control 6", y=T33."High Res Display") -> (x = y?=w3252:bool)
    n2428 = Multiply(x=10.0, y=w3129) -> (x*y=→"Trap 1 Position RMS (A)":dbl)
    n2429 = case "For displaying the high resolution display (no downsampling)" shown="True" w3252 {
      tunnel: w3218 -> [_ w3578]
      frame False {
      }
      frame True {
        n2430 = Index Array(array=w3578, index="High Res. Display") -> (element=w3579:waveform(dbl))
        n2431 = call <vilib>:"Std Deviation and Variance.vi"("X"=w3579) -> ("mean"=w3586:dbl, "standard deviation"=w3591:dbl)  [unwired: 1 in, 1 out]
        "Mean Intensity" <- w3586
        "Sigma" <- w3591
        n2432 = Subtract(x=w3579, y=w3586) -> (x-y=w3585:waveform(dbl))
        n2433 = Select(t=w3585, s="Subtract mean", f=w3579) -> (s? t:f=→"1 Channel":waveform(dbl))
        n2434 = Divide(x=w3591, y=w3586) -> (x/y=→"Sigma/Mean":dbl)
        n2435 = feedback #9(1) -> (w3580:i32)
        n2436 = Greater Or Equal?(x=w3580, y="Slow mean N ave.") -> (x >= y?=w3593:bool)
        n2437 = Increment(x=w3580) -> (x+1=w3595:i32)
        n2438 = Select(t=1, s=w3593, f=w3595) -> (s? t:f=w3582:i32)
        n2439 = feedback-in #9(w3582) -> ()
        n2440 = feedback #10() -> (w3583:waveform(dbl))  [unwired: 1 out]
        n2441 = case shown="Default" w3580 {
          tunnel: [w3598 w3601] -> w3584
          tunnel: w3583 -> [w3600 _]
          tunnel: w3579 -> [w3599 w3601]
          frame Default {
            n2442 = call-poly <vilib>:"Append Waveforms.vi"("waveform B"=w3599, "waveform A"=w3600) -> ("waveform out"=w3598:waveform(dbl))  [unwired: 1 in, 8 out]
          }
          frame 1 {
          }
        }
        n2443 = feedback-in #10(w3584) -> ()
        n2444 = case shown="True" w3593 {
          tunnel: w3584 -> [_ w3597]
          frame False {
          }
          frame True {
            n2445 = call-poly <vilib>:"Mean.vi"("X"=w3597) -> ("mean"=→"Slow mean":dbl)  [unwired: 1 out]
          }
        }
      }
    }
    n2446 = case "For plotting results of scanning MCL (fluorescence and detection laser images)" shown="True" w3320 {
      tunnel: w3319 -> [_ w3710]
      tunnel: w3328 -> [_ _]
      tunnel: w3218 -> [_ w3840]
      tunnel: w3196 -> [_ w3748]
      tunnel: w3039 -> [_ w3717]
      frame False {
      }
      frame True {
        w3727 = u32 0 items=["Horizontal", "Vertical", "Central", "1st Diagonal", "2nd Diagonal"] ("Type of Symmetry")
        w3755 = u32 0 items=["Horizontal", "Vertical", "Central", "1st Diagonal", "2nd Diagonal"] ("Type of Symmetry")
        w3779 = u32 0 items=["Horizontal", "Vertical", "Central", "1st Diagonal", "2nd Diagonal"] ("Type of Symmetry")
        w3782 = u32 0 items=["Horizontal", "Vertical", "Central", "1st Diagonal", "2nd Diagonal"] ("Type of Symmetry")
        w3811 = u32 0 items=["Horizontal", "Vertical", "Central", "1st Diagonal", "2nd Diagonal"] ("Type of Symmetry")
        n2447 = Unbundle(w3717) -> (w3716:u32[], w3714:u32[], w3712:u32[])
        n2448 = To Double Precision Float(number=w3716) -> (double precision float=w3715:dbl[])
        n2449 = To Double Precision Float(number=w3714) -> (double precision float=w3713:dbl[])
        n2450 = To Double Precision Float(number=w3712) -> (double precision float=w3711:dbl[])
        n2451 = Index Array(array=w3840, index=10) -> (element=w3846:waveform(dbl))
        n2452 = Index Array(array=w3840, index=11) -> (element=w3843:waveform(dbl))
        n2453 = local read "Cycles/step (MCL)"() -> (w3796:u64)
        n2454 = Index Array(array=w3840, index="Channel") -> (element=w3842:waveform(dbl))
        n2455 = Unbundle(w3748) -> ("New Image"=w3747:T2, "New Image"=w3746:T2, "New Image"=w3718:T2, "New Image"=w3719:T2, "New Image"=w3720:T2)
        n2456 = local read "Scan steps (MCL)"() -> (w3706:u64)
        n2457 = Unbundle By Name(w3846) -> ("Y"=w3798:dbl[])
        n2458 = Unbundle By Name(w3843) -> ("Y"=w3800:dbl[])
        n2459 = local read "Scan lines (y)"() -> (w3707:u64)
        n2460 = local read "N APD Samp/step"() -> (w3709:dbl)
        n2461 = Unbundle By Name(w3842) -> ("Y"=w3805:dbl[])
        n2462 = call "downsample 1D array - double.vi"("Ave N"=w3796, "Array In"=w3798) -> ("Array Out"=w3797:dbl[])  [unwired: 1 out]
        n2463 = call "downsample 1D array - double.vi"("Ave N"=w3796, "Array In"=w3800) -> ("Array Out"=w3799:dbl[])  [unwired: 1 out]
        n2464 = call "downsample 1D array - double.vi"("Ave N"=w3796, "Array In"=w3805) -> ("Array Out"=w3804:dbl[])  [unwired: 1 out]
        n2465 = Multiply(x=w3706, y=u64 2) -> (x*y=w3708:u64)
        n2466 = feedback #11(w3713) -> (w3773:dbl[])
        n2467 = Build Array (concatenate)(w3773, w3713) -> (w3772:dbl[])
        n2468 = feedback #12(w3711) -> (w3745:dbl[])